vi "Velociprobe_Nanopositioner_Control_RT 2c.vi"() -> ()   [LabVIEW 2015] (continued)
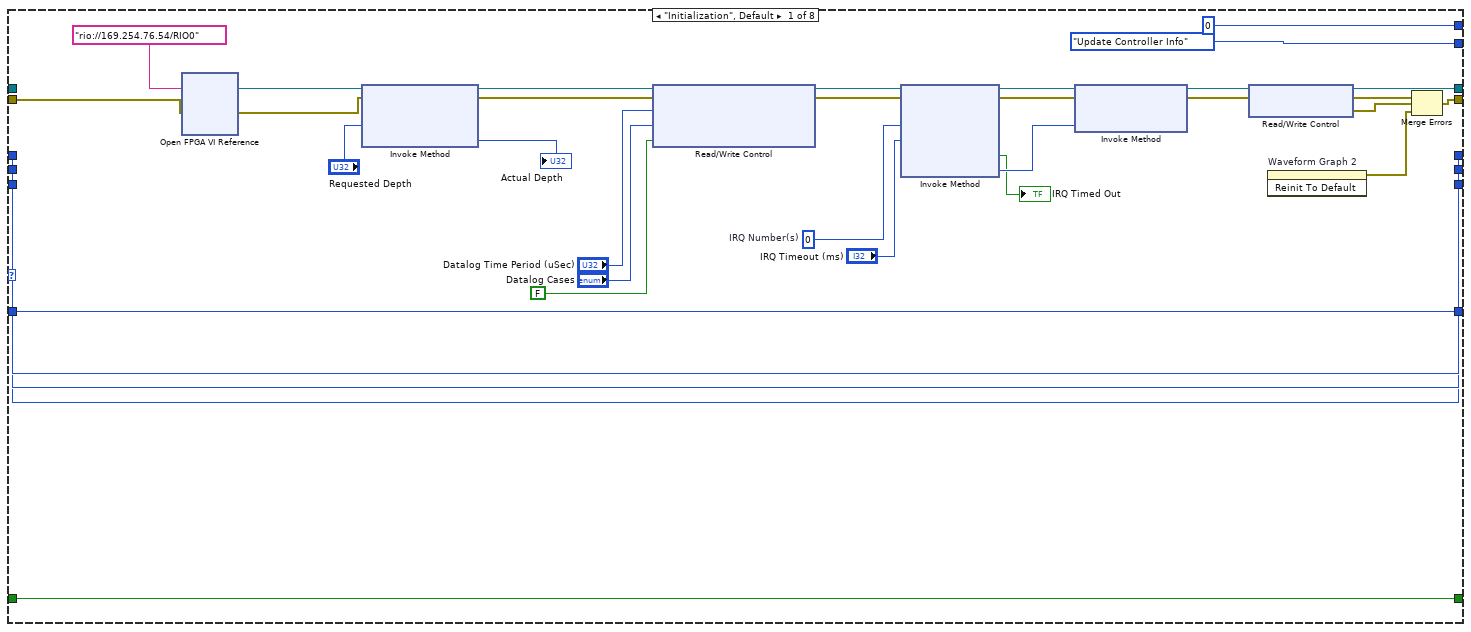
[diagram p2: hidden frame]
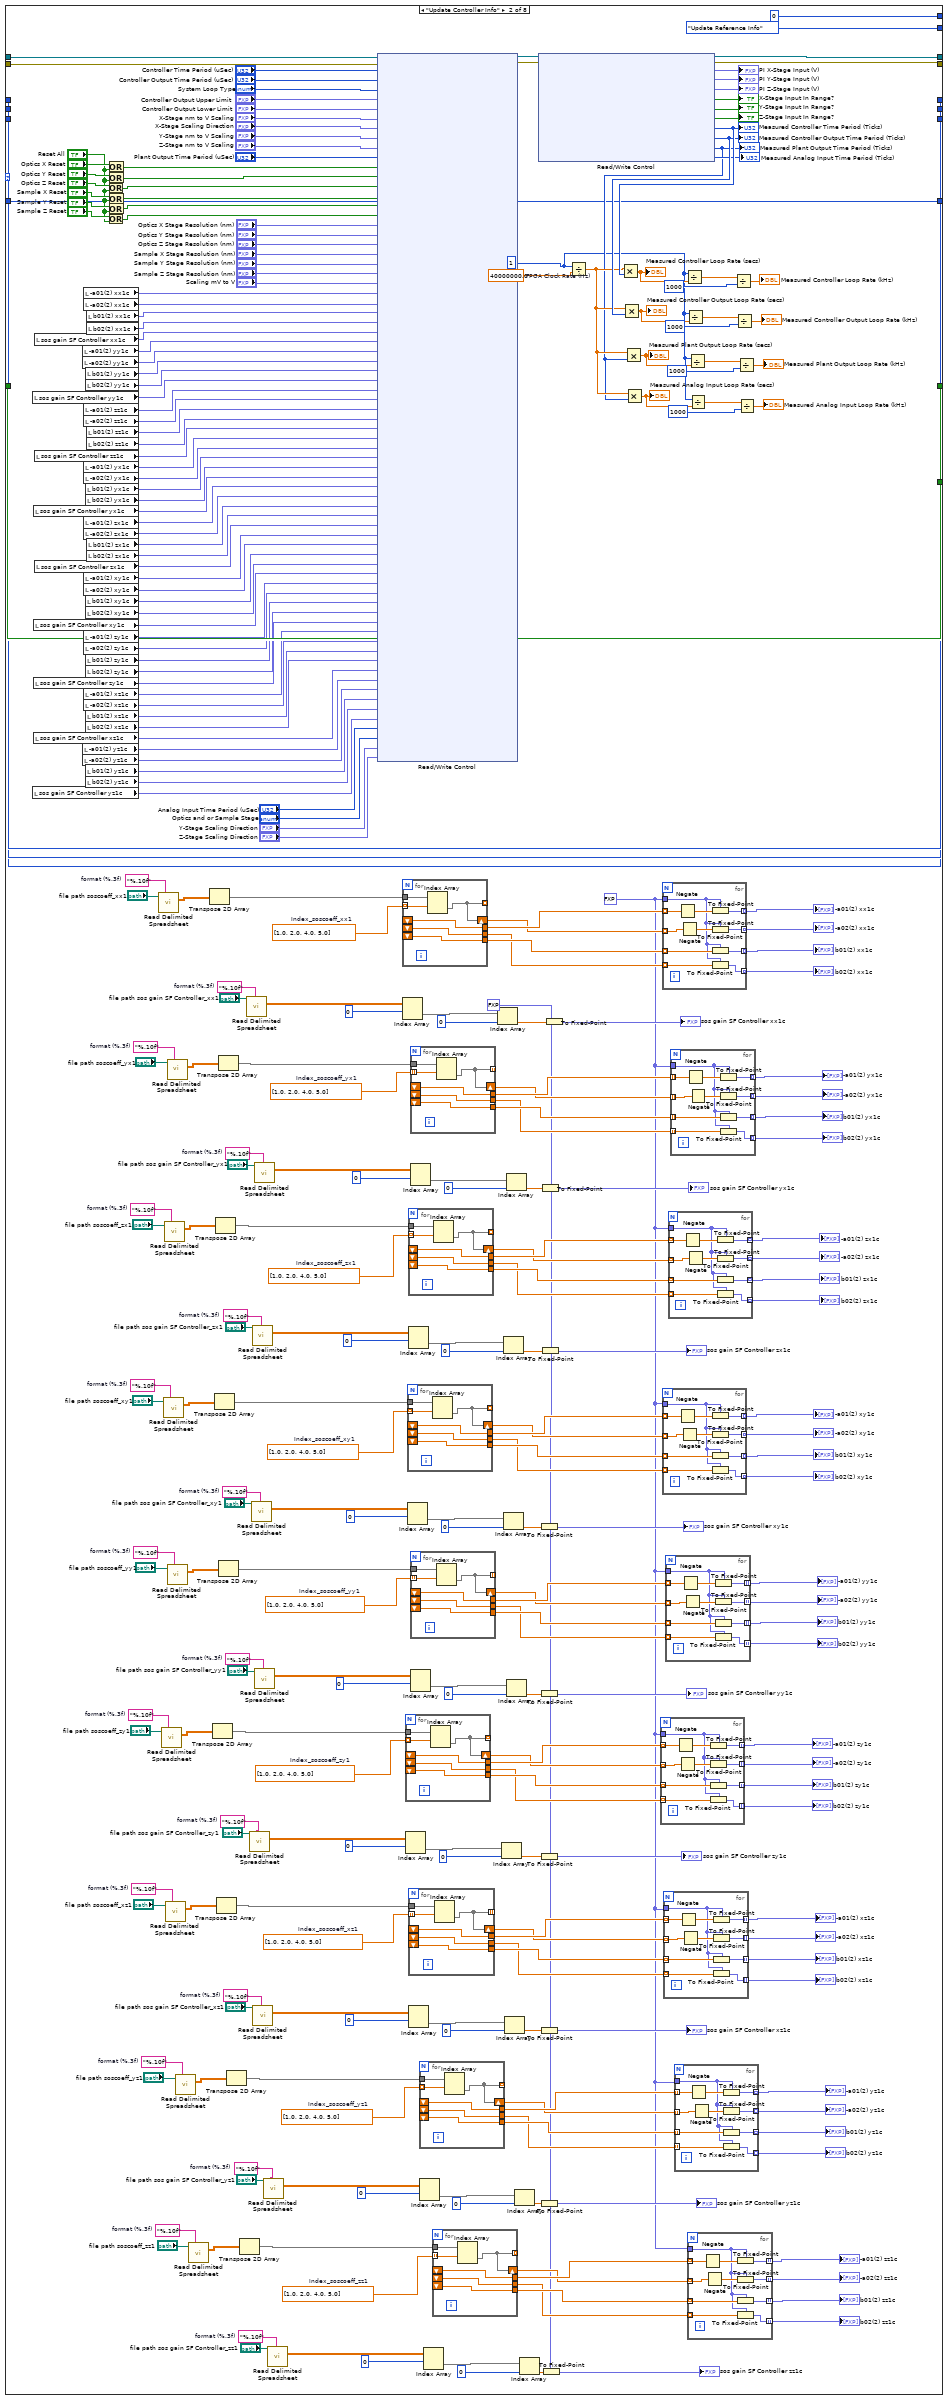
[diagram p3: hidden frame]
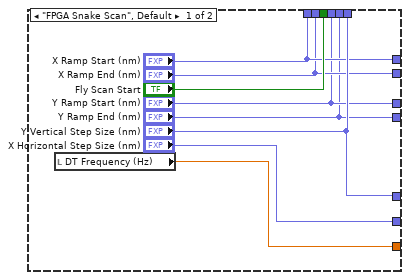
[diagram p4: hidden frame]
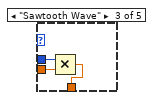
[diagram p6: hidden frame]
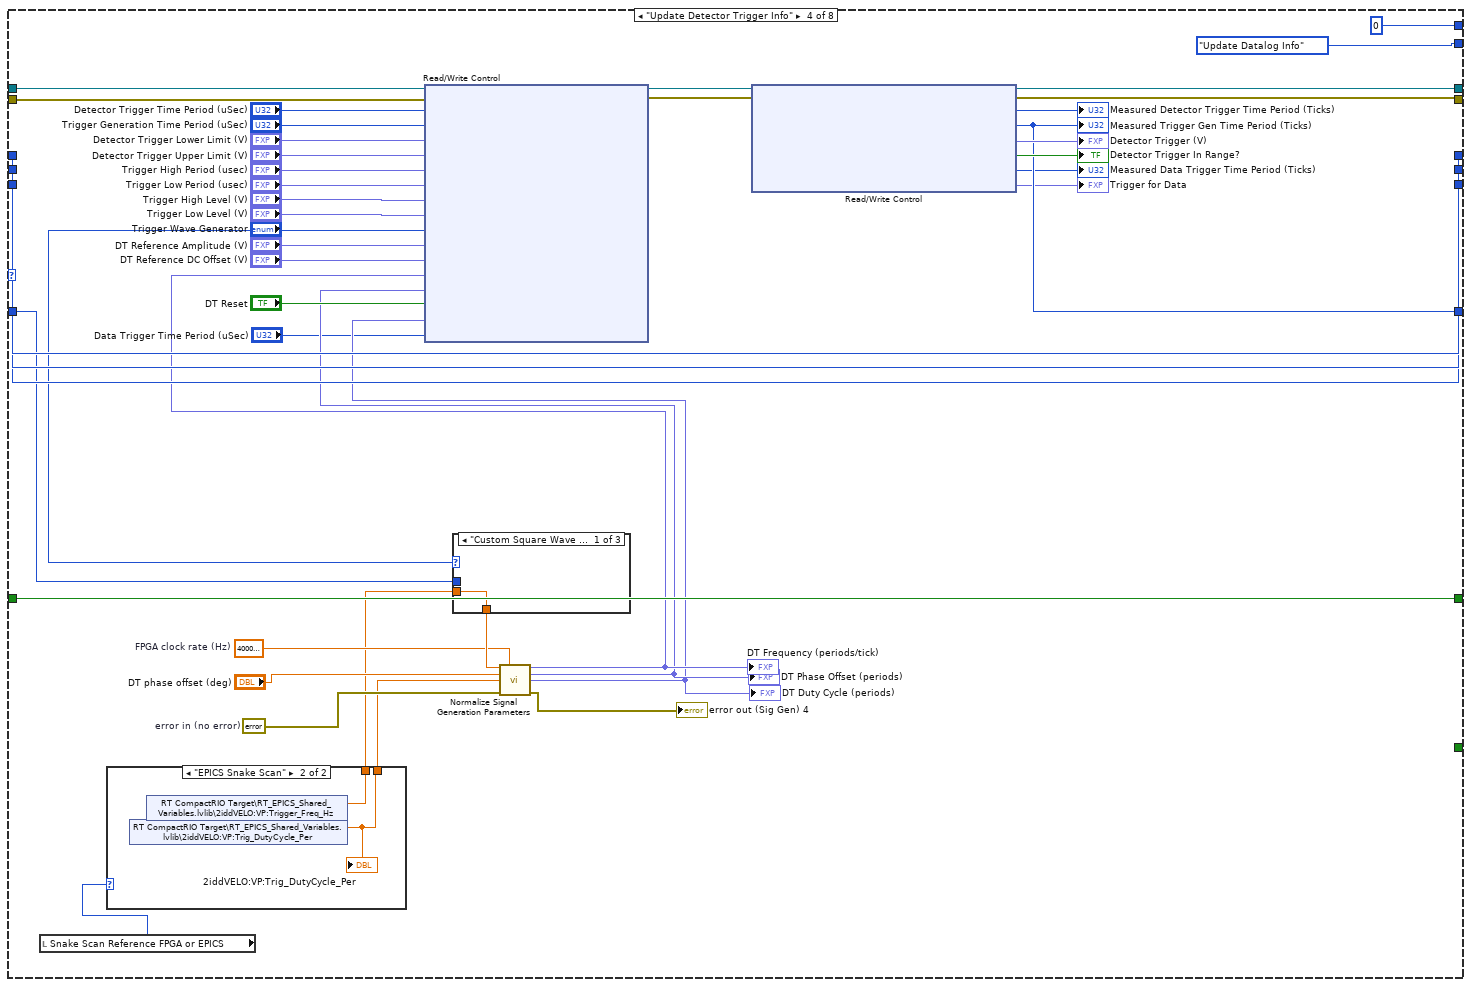
[diagram p15: hidden frame]
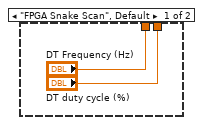
[diagram p16: hidden frame]
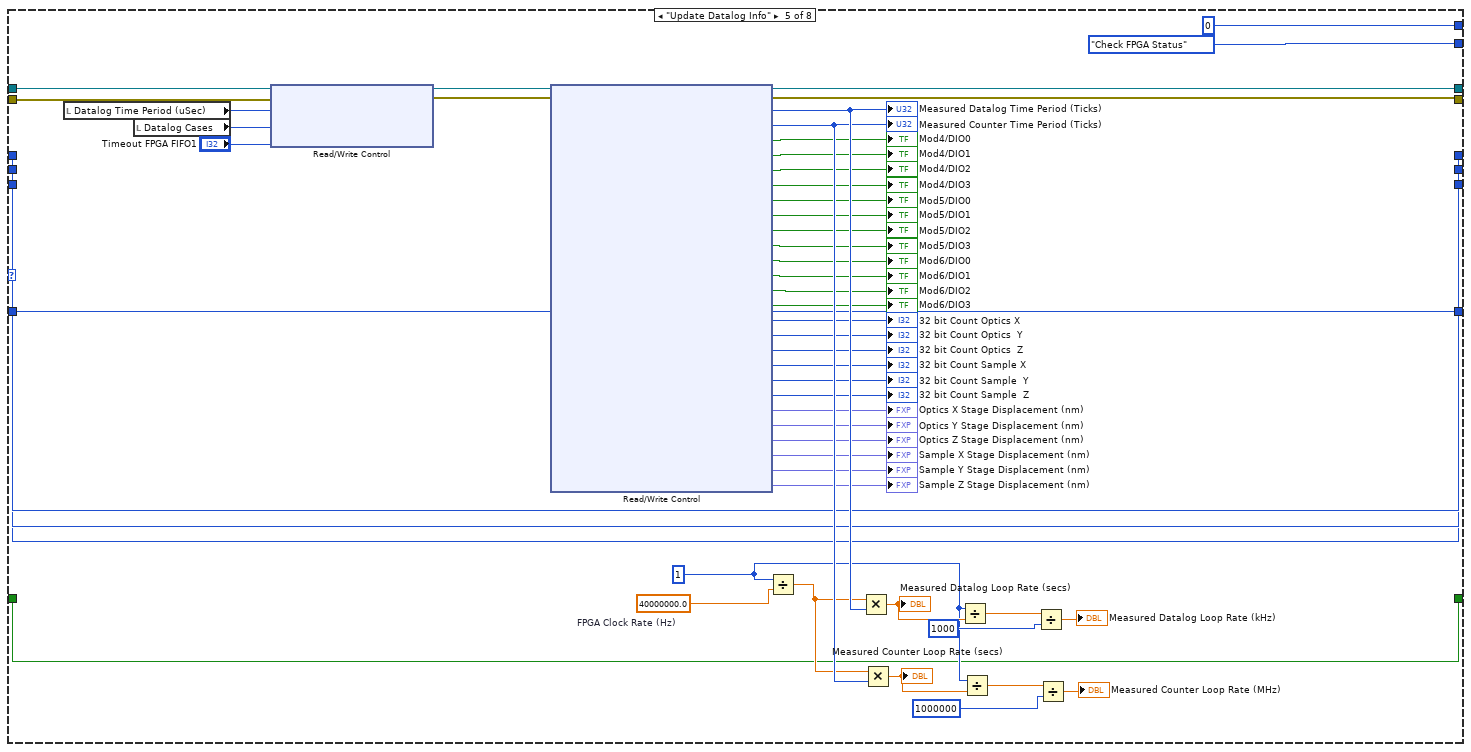
[diagram p19: hidden frame]
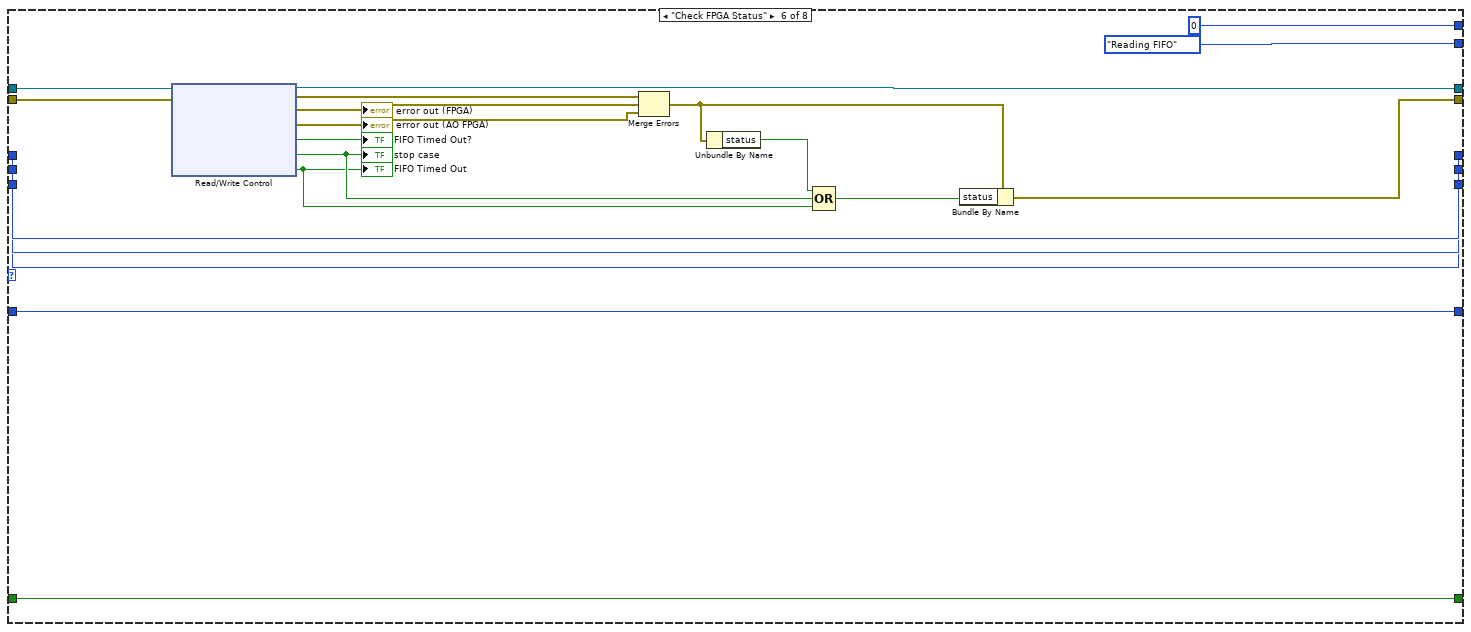
[diagram p20: hidden frame]
        }
        "-a01(2) zz1c" <- w292
        "-a02(2) zz1c" <- w291
        "b01(2) zz1c" <- w290
        "b02(2) zz1c" <- w289
        n211 = Divide(x=w81, y=w87) -> (x/y=w86:dbl)
        n212 = Divide(x=w362, y=1000) -> (x/y=→"Measured Controller Loop Rate (kHz)":dbl)
        n213 = Divide(x=w358, y=1000) -> (x/y=→"Measured Controller Output Loop Rate (kHz)":dbl)
        n214 = Divide(x=w354, y=1000) -> (x/y=→"Measured Plant Output Loop Rate (kHz)":dbl)
        n215 = Divide(x=w86, y=1000) -> (x/y=→"Measured Analog Input Loop Rate (kHz)":dbl)
      }
      frame "Update Reference Info" {
        w607 = 40000000.0  # FPGA Clock Rate (Hz)
        w601 = 1
        w614 = 40000000.0  # FPGA Clock Rate (Hz)
        w608 = 1
        w619 = errorcluster {"status"=FALSE, "code"=0, "source"=""}  # error in (no error)
        w622 = errorcluster {"status"=FALSE, "code"=0, "source"=""}  # error in (no error)
        w636 = 40000000.0  # FPGA Clock Rate (Hz)
        w630 = 1
        w648 = errorcluster {"status"=FALSE, "code"=0, "source"=""}  # error in (no error)
        w615 = 40000000.0  # FPGA clock rate (Hz)
        n216 = case shown="\"EPICS Snake Scan\"" "Snake Scan Reference FPGA or EPICS" {
          tunnel: ["X Ramp Start (nm)" w666] -> w548
          tunnel: ["X Ramp End (nm)" w665] -> w547
          tunnel: ["Fly Scan Start" w671] -> w546
          tunnel: ["Y Ramp Start (nm)" w664] -> w545
          tunnel: ["Y Ramp End (nm)" w663] -> w544
          tunnel: ["Y Vertical Step Size (nm)" w667] -> w543
          tunnel: ["X Horizontal Step Size (nm)" w670] -> w542
          tunnel: [w657 w668] -> w541
          tunnel: ["Y Vertical Step Size (nm)" w667] -> w534
          tunnel: ["X Ramp Start (nm)" w666] -> w533
          tunnel: ["X Ramp End (nm)" w665] -> w532
          tunnel: ["Y Ramp Start (nm)" w664] -> w531
          tunnel: ["Y Ramp End (nm)" w663] -> w530
          frame "FPGA Snake Scan", Default {
            n217 = local read "DT Frequency (Hz)"() -> (w657:dbl)
          }
          frame "EPICS Snake Scan" {
            w669 = fxp<+/-,16,16> 0.0 ("fixed-point type")
            n218 = shared-variable "RT CompactRIO Target\\RT_EPICS_Shared_Variables.lvlib\\2iddVELO:VP:Trigger_Freq_Hz"() -> (w668:dbl)  [unwired: 1 in, 1 out]
            "2iddVELO:VP:Trigger_Freq_Hz" <- w668
            n219 = shared-variable "RT CompactRIO Target\\RT_EPICS_Shared_Variables.lvlib\\2iddVELO:VP:Y_Step_Size_nm"() -> (w673:dbl)  [unwired: 1 in, 1 out]
            "2iddVELO:VP:Y_Step_Size_nm" <- w673
            n220 = shared-variable "RT CompactRIO Target\\RT_EPICS_Shared_Variables.lvlib\\2iddVELO:VP:X_Step_Size_nm"() -> (w672:dbl)  [unwired: 1 in, 1 out]
            "2iddVELO:VP:X_Step_Size_nm" <- w672
            n221 = shared-variable "RT CompactRIO Target\\RT_EPICS_Shared_Variables.lvlib\\2iddVELO:VP:Y_Start_nm"() -> (w674:dbl)  [unwired: 1 in, 1 out]
            n222 = shared-variable "RT CompactRIO Target\\RT_EPICS_Shared_Variables.lvlib\\2iddVELO:VP:Y_End_nm"() -> (w662:dbl)  [unwired: 1 in, 1 out]
            n223 = shared-variable "RT CompactRIO Target\\RT_EPICS_Shared_Variables.lvlib\\2iddVELO:VP:Flyscan_Start"() -> (w671:bool)  [unwired: 1 in, 1 out]
            "2iddVELO:VP:Flyscan_Start" <- w671
            n224 = shared-variable "RT CompactRIO Target\\RT_EPICS_Shared_Variables.lvlib\\2iddVELO:VP:X_Start_nm"() -> (w676:dbl)  [unwired: 1 in, 1 out]
            "2iddVELO:VP:X_Start_nm" <- w676
            n225 = shared-variable "RT CompactRIO Target\\RT_EPICS_Shared_Variables.lvlib\\2iddVELO:VP:X_End_nm"() -> (w675:dbl)  [unwired: 1 in, 1 out]
            "2iddVELO:VP:X_End_nm" <- w675
            n226 = Negate(x=w662) -> (-x=w661:dbl)
            "2iddVELO:VP:Y_End_nm" <- w661
            n227 = Negate(x=w674) -> (-x=w660:dbl)
            "2iddVELO:VP:Y_Start_nm" <- w660
            n228 = To Fixed-Point(fixed-point type=w669, number=w676) -> (fixed-point=w666:fxp<+/-,16,16>)
            n229 = To Fixed-Point(fixed-point type=w669, number=w675) -> (fixed-point=w665:fxp<+/-,16,16>)
            n230 = To Fixed-Point(fixed-point type=w669, number=w660) -> (fixed-point=w664:fxp<+/-,16,16>)
            n231 = To Fixed-Point(fixed-point type=w669, number=w661) -> (fixed-point=w663:fxp<+/-,16,16>)
            n232 = To Fixed-Point(fixed-point type=w669, number=w673) -> (fixed-point=w667:fxp<+/-,16,16>)
            n233 = To Fixed-Point(fixed-point type=w669, number=w672) -> (fixed-point=w670:fxp<+/-,16,16>)
          }
        }
        n234 = local read "X Ramp Period (usec)"() -> (w550:fxp<+,24,24>)
        n235 = local read "Y Ramp Period (usec)"() -> (w551:fxp<+,24,24>)
        n236 = case shown="\"Constant\", Default" "Z Reference Wave Selection" {
          tunnel: "Z frequency (Hz)" -> [w677 w678 w680 w682 w683]
          tunnel: [w677 w678 w679 w682 w683] -> w576
          tunnel: w575 -> [_ _ w681 _ _]
          frame "Constant", Default {
          }
          frame "Sine Wave" {
          }
          frame "Sawtooth Wave" {
            n237 = Multiply(x=w681, y=w680) -> (x*y=w679:dbl)
          }
          frame "Square Wave" {
          }
          frame "Filtered White Noise" {
          }
        }
        n238 = case shown="\"Constant\", Default" "Y Reference Wave Selection" {
          tunnel: "Y frequency (Hz)" -> [w684 w685 w686 w687]
          tunnel: [w684 w685 w686 w687] -> w581
          tunnel: w578 -> [_ _ _ _]
          frame "Constant", Default {
          }
          frame "Sine Wave" {
          }
          frame "Custom Ramp Wave" {
          }
          frame "Filtered White Noise" {
          }
        }
        n239 = case shown="\"Custom Up Down Ramp\"" "X Reference Wave Selection" {
          tunnel: "X frequency (Hz)" -> [w688 w689 w690 w691]
          tunnel: [w688 w689 w690 w691] -> w585
          tunnel: w583 -> [_ _ _ _]
          frame "Constant", Default {
          }
          frame "Sine Wave" {
          }
          frame "Custom Up Down Ramp" {
          }
          frame "Filtered White Noise" {
          }
        }
        n240 = call <vilib>:"Normalize Signal Generation Parameters.vi"("frequency (Hz)"=w581, "FPGA clock rate (Hz)"=w615, "phase offset (deg)"="Y phase offset (deg)", "error in (no error)"=w622) -> ("frequency (periods/tick)"=w618:fxp<+,32,0>, "phase offset (periods)"=w617:fxp<+,32,0>, "error out"=→"error out (Sig Gen) 2":errorcluster)  [unwired: 6 in, 3 out]
        "Y frequency (periods/tick)" <- w618
        "Y phase offset (periods)" <- w617
        n241 = call <vilib>:"Normalize Signal Generation Parameters.vi"("frequency (Hz)"=w576, "FPGA clock rate (Hz)"=w615, "phase offset (deg)"="Z phase offset (deg)", "error in (no error)"=w619) -> ("frequency (periods/tick)"=w616:fxp<+,32,0>, "phase offset (periods)"=w594:fxp<+,32,0>, "error out"=→"error out (Sig Gen) 3":errorcluster)  [unwired: 6 in, 3 out]
        "Z frequency (periods/tick)" <- w616
        "Z phase offset (periods)" <- w594
        n242 = call <vilib>:"Normalize Signal Generation Parameters.vi"("frequency (Hz)"=w585, "FPGA clock rate (Hz)"=w615, "phase offset (deg)"="X phase offset (deg)", "error in (no error)"=w648) -> ("frequency (periods/tick)"=w647:fxp<+,32,0>, "phase offset (periods)"=w625:fxp<+,32,0>, "error out"=→"error out (Sig Gen)":errorcluster)  [unwired: 6 in, 3 out]
        "X frequency (periods/tick)" <- w647
        "X phase offset (periods)" <- w625
        n243 = xnode "Read/Write Control"("FPGA VI Reference In"=w540, "error in"=w539, "X Reference Time Period (uSec)"="X Reference Time Period (uSec)", "Y Reference Time Period (uSec)"="Y Reference Time Period (uSec)", "Z Reference Time Period (uSec)"="Z Reference Time Period (uSec)", "X Reference Wave Selection"="X Reference Wave Selection", "Y Reference Wave Selection"="Y Reference Wave Selection", "Z Reference Wave Selection"="Z Reference Wave Selection", "X Reference Reset"="X Reference Reset", "Y Reference Reset"="Y Reference Reset", "Z Reference Reset"="Z Reference Reset", "X Reference Amplitude (nm)"="X Reference Amplitude (nm)", "Y Reference Amplitude (nm)"="Y Reference Amplitude (nm)", "Z Reference Amplitude (nm)"="Z Reference Amplitude (nm)", "X Frequency (periods/tick)"=w647, "X Phase Offset (periods)"=w625, "Y Frequency (periods/tick)"=w618, "Y Phase Offset (periods)"=w617, "Z Frequency (periods/tick)"=w616, "Z Phase Offset (periods)"=w594, "X Reference DC Offset (nm)"="X Reference DC Offset (nm)", "Y Reference DC Offset (nm)"="Y Reference DC Offset (nm)", "Z Reference DC Offset (nm)"="Z Reference DC Offset (nm)", "X White Noise Amplitude"="X White Noise Amplitude", "X White Noise Seed"="X White Noise Seed", "Y White Noise Amplitude"="Y White Noise Amplitude", "Y White Noise Seed"="Y White Noise Seed", "Z White Noise Amplitude"="Z White Noise Amplitude", "Z White Noise Seed"="Z White Noise Seed", "Mod 3 AI0 V to nm Scaling"="Mod 3 AI0 V to nm Scaling", "Mod 3 AI1 V to nm Scaling"="Mod 3 AI1 V to nm Scaling", "Mod 3 AI2 V to nm Scaling"="Mod 3 AI2 V to nm Scaling", "X Ramp Period (usec)"=w550, "X Ramp Start (nm)"=w548, "X Ramp End (nm)"=w547, "X Start Marker (nm)"="X Start Marker (nm)", "Fly Scan Start"=w546, "Y Ramp Period (usec)"=w551, "Y Ramp Start (nm)"=w545, "Y Ramp End (nm)"=w544, "Y Ramp Drop Size (nm)"=w543, "Y Start Marker (nm)"="Y Start Marker (nm)") -> ("FPGA VI Reference Out"=w538:refnum<k20>, "error out"=w537:errorcluster)
        n244 = xnode "Read/Write Control"("FPGA VI Reference In"=w538, "error in"=w537) -> ("FPGA VI Reference Out"=w535:refnum<k20>, "error out"=w536:errorcluster, "X Stage Reference (nm)"=→"X Stage Reference (nm)":fxp<+/-,58,25>, "Y Stage Reference (nm)"=→"Y Stage Reference (nm)":fxp<+/-,58,25>, "Z Stage Reference (nm)"=→"Z Stage Reference (nm)":fxp<+/-,58,25>, "Measured X Reference Time Period (Ticks)"=w584:u32, "Measured Y Reference Time Period (Ticks)"=w580:u32, "Measured Z Reference Time Period (Ticks)"=w579:u32, "Fly Scan Running"=→"Fly Scan Running":bool, "Continue Run"=→"Continue Run":bool)
        "Measured X Reference Time Period (Ticks)" <- w584
        "Measured Y Reference Time Period (Ticks)" <- w580
        "Measured Z Reference Time Period (Ticks)" <- w579
        n245 = Subtract(x=w531, y=w530) -> (x-y=w567:fxp<+/-,17,17>)
        n246 = Subtract(x=w533, y=w532) -> (x-y=w565:fxp<+/-,17,17>)
        n247 = Absolute Value(x=w567) -> (abs(x)=w558:fxp<+,16,16>)
        n248 = Absolute Value(x=w565) -> (abs(x)=w564:fxp<+,16,16>)
        n249 = Divide(x=w564, y=w542) -> (x/y=w562:fxp<+/-,33,17>)
        "# of Points per Line" <- w562
        n250 = Divide(x=w630, y=w636) -> (x/y=w631:dbl)
        n251 = Divide(x=w608, y=w614) -> (x/y=w609:dbl)
        n252 = Divide(x=w601, y=w607) -> (x/y=w602:dbl)
        n253 = Divide(x=w562, y=w541) -> (x/y=w554:dbl)
        "sec per line" <- w554
        n254 = Multiply(x=w631, y=w584) -> (x*y=w635:dbl)
        "Measured X Reference Loop Rate (secs)" <- w635
        n255 = Multiply(x=w609, y=w580) -> (x*y=w613:dbl)
        "Measured Y Reference Loop Rate (secs)" <- w613
        n256 = Divide(x=w558, y=w534) -> (x/y=w559:fxp<+/-,33,17>)
        n257 = Multiply(x=w602, y=w579) -> (x*y=w606:dbl)
        "Measured Z Reference Loop Rate (secs)" <- w606
        n258 = Add(x=w559, y=fxp<+,16,16> 1.0) -> (x+y=w553:fxp<+/-,34,18>)
        "# of Hor Lines" <- w553
        n259 = Multiply(x=w554, y=1000000.0) -> (x*y=w557:dbl)
        "X Ramp Period DBL (usec)" <- w557
        n260 = Reciprocal(x=w554) -> (1/x=→"line per sec (Hz)":dbl)
        n261 = Divide(x=w630, y=w635) -> (x/y=w634:dbl)
        n262 = Divide(x=w608, y=w613) -> (x/y=w612:dbl)
        n263 = To Fixed-Point(fixed-point type=fxp<+,24,24> 0.0, number=w557) -> (fixed-point=→"X Ramp Period (usec)" →"Y Ramp Period (usec)":fxp<+,24,24>)
        n264 = Multiply(x=w554, y=w553) -> (x*y=→"Total Scan Time (sec)":dbl)
        n265 = Divide(x=w601, y=w606) -> (x/y=w605:dbl)
        n266 = Multiply(x=w553, y=w562) -> (x*y=→"# Total Trigger Points":fxp<+/-,64,34>)
        n267 = Divide(x=w634, y=1000) -> (x/y=→"Measured X Reference Loop Rate (kHz)":dbl)
        n268 = Divide(x=w612, y=1000) -> (x/y=→"Measured Y Reference Loop Rate (kHz)":dbl)
        n269 = Divide(x=w605, y=1000) -> (x/y=→"Measured Z Reference Loop Rate (kHz)":dbl)
      }
      frame "Update Detector Trigger Info" {
        w710 = 40000000.0  # FPGA clock rate (Hz)
        w712 = errorcluster {"status"=FALSE, "code"=0, "source"=""}  # error in (no error)
        n270 = local read "Snake Scan Reference FPGA or EPICS"() -> (w703:enum16{"FPGA Snake Scan", "EPICS Snake Scan"})
        n271 = case shown="\"EPICS Snake Scan\"" w703 {
          tunnel: ["DT Frequency (Hz)" w738] -> w702
          tunnel: ["DT duty cycle (%)" w737] -> w701
          frame "FPGA Snake Scan", Default {
          }
          frame "EPICS Snake Scan" {
            n272 = shared-variable "RT CompactRIO Target\\RT_EPICS_Shared_Variables.lvlib\\2iddVELO:VP:Trig_DutyCycle_Per"() -> (w737:dbl)  [unwired: 1 in, 1 out]
            "2iddVELO:VP:Trig_DutyCycle_Per" <- w737
            n273 = shared-variable "RT CompactRIO Target\\RT_EPICS_Shared_Variables.lvlib\\2iddVELO:VP:Trigger_Freq_Hz"() -> (w738:dbl)  [unwired: 1 in, 1 out]
          }
        }
        n274 = case shown="\"Custom Square Wave \", Default" "Trigger Wave Generator" {
          tunnel: w702 -> [w739 w740 w741]
          tunnel: [w739 w740 w741] -> w711
          tunnel: w704 -> [_ _ _]
          frame "Custom Square Wave ", Default {
          }
          frame "Square Wave 1" {
          }
          frame "Square Wave 2" {
          }
        }
        n275 = call <vilib>:"Normalize Signal Generation Parameters.vi"("frequency (Hz)"=w711, "FPGA clock rate (Hz)"=w710, "phase offset (deg)"="DT phase offset (deg)", "duty cycle (%)"=w701, "error in (no error)"=w712) -> ("frequency (periods/tick)"=w708:fxp<+,32,0>, "phase offset (periods)"=w707:fxp<+,32,0>, "duty cycle (periods)"=w706:fxp<+,32,0>, "error out"=→"error out (Sig Gen) 4":errorcluster)  [unwired: 5 in, 2 out]
        "DT Frequency (periods/tick)" <- w708
        "DT Phase Offset (periods)" <- w707
        "DT Duty Cycle (periods)" <- w706
        n276 = xnode "Read/Write Control"("FPGA VI Reference In"=w700, "error in"=w699, "Detector Trigger Time Period (uSec)"="Detector Trigger Time Period (uSec)", "Trigger Generation Time Period (uSec)"="Trigger Generation Time Period (uSec)", "Detector Trigger Lower Limit (V)"="Detector Trigger Lower Limit (V)", "Detector Trigger Upper Limit (V)"="Detector Trigger Upper Limit (V)", "Trigger High Period (usec)"="Trigger High Period (usec)", "Trigger Low Period (usec)"="Trigger Low Period (usec)", "Trigger High Level (V)"="Trigger High Level (V)", "Trigger Low Level (V)"="Trigger Low Level (V)", "Trigger Wave Generator"="Trigger Wave Generator", "DT Reference Amplitude (V)"="DT Reference Amplitude (V)", "DT Reference DC Offset (V)"="DT Reference DC Offset (V)", "DT Frequency (periods/tick)"=w708, "DT Phase Offset (periods)"=w707, "DT Reset"="DT Reset", "DT Duty Cycle (periods)"=w706, "Data Trigger Time Period (uSec)"="Data Trigger Time Period (uSec)") -> ("FPGA VI Reference Out"=w698:refnum<k20>, "error out"=w697:errorcluster)
        n277 = xnode "Read/Write Control"("FPGA VI Reference In"=w698, "error in"=w697) -> ("FPGA VI Reference Out"=w696:refnum<k20>, "error out"=w695:errorcluster, "Measured Detector Trigger Time Period (Ticks)"=→"Measured Detector Trigger Time Period (Ticks)":u32, "Measured Trigger Gen Time Period (Ticks)"=w705:u32, "Detector Trigger (V)"=→"Detector Trigger (V)":fxp<+/-,20,5>, "Detector Trigger In Range?"=→"Detector Trigger In Range?":bool, "Measured Data Trigger Time Period (Ticks)"=→"Measured Data Trigger Time Period (Ticks)":u32, "Trigger for Data"=→"Trigger for Data":fxp<+/-,58,25>)
        "Measured Trigger Gen Time Period (Ticks)" <- w705
      }
      frame "Update Datalog Info" {
        w786 = 40000000.0  # FPGA Clock Rate (Hz)
        w775 = 1
        n278 = local read "Datalog Time Period (uSec)"() -> (w773:u32)
        n279 = local read "Datalog Cases"() -> (w772:T6)
        n280 = xnode "Read/Write Control"("FPGA VI Reference In"=w747, "error in"=w746, "Datalog Time Period (uSec)"=w773, "Datalog Cases"=w772, "Timeout FPGA FIFO1"="Timeout FPGA FIFO1") -> ("FPGA VI Reference Out"=w745:refnum<k20>, "error out"=w744:errorcluster)
        n281 = xnode "Read/Write Control"("FPGA VI Reference In"=w745, "error in"=w744) -> ("FPGA VI Reference Out"=w742:refnum<k20>, "error out"=w743:errorcluster, "Measured Datalog Time Period (Ticks)"=w785:u32, "Measured Counter Time Period (Ticks)"=w783:u32, "Mod4/DIO0"=→"Mod4/DIO0":bool, "Mod4/DIO1"=→"Mod4/DIO1":bool, "Mod4/DIO2"=→"Mod4/DIO2":bool, "Mod4/DIO3"=→"Mod4/DIO3":bool, "Mod5/DIO0"=→"Mod5/DIO0":bool, "Mod5/DIO1"=→"Mod5/DIO1":bool, "Mod5/DIO2"=→"Mod5/DIO2":bool, "Mod5/DIO3"=→"Mod5/DIO3":bool, "Mod6/DIO0"=→"Mod6/DIO0":bool, "Mod6/DIO1"=→"Mod6/DIO1":bool, "Mod6/DIO2"=→"Mod6/DIO2":bool, "Mod6/DIO3"=→"Mod6/DIO3":bool, "32 bit Count Optics X"=→"32 bit Count Optics X":i32, "32 bit Count Optics  Y"=→"32 bit Count Optics  Y":i32, "32 bit Count Optics  Z"=→"32 bit Count Optics  Z":i32, "32 bit Count Sample X"=→"32 bit Count Sample X":i32, "32 bit Count Sample  Y"=→"32 bit Count Sample  Y":i32, "32 bit Count Sample  Z"=→"32 bit Count Sample  Z":i32, "Optics X Stage Displacement (nm)"=→"Optics X Stage Displacement (nm)":fxp<+/-,58,25>, "Optics Y Stage Displacement (nm)"=→"Optics Y Stage Displacement (nm)":fxp<+/-,58,25>, "Optics Z Stage Displacement (nm)"=→"Optics Z Stage Displacement (nm)":fxp<+/-,58,25>, "Sample X Stage Displacement (nm)"=→"Sample X Stage Displacement (nm)":fxp<+/-,58,25>, "Sample Y Stage Displacement (nm)"=→"Sample Y Stage Displacement (nm)":fxp<+/-,58,25>, "Sample Z Stage Displacement (nm)"=→"Sample Z Stage Displacement (nm)":fxp<+/-,58,25>)
        "Measured Datalog Time Period (Ticks)" <- w785
        "Measured Counter Time Period (Ticks)" <- w783
        n282 = Divide(x=w775, y=w786) -> (x/y=w782:dbl)
        n283 = Multiply(x=w782, y=w785) -> (x*y=w793:dbl)
        "Measured Datalog Loop Rate (secs)" <- w793
        n284 = Multiply(x=w782, y=w783) -> (x*y=w789:dbl)
        "Measured Counter Loop Rate (secs)" <- w789
        n285 = Divide(x=w775, y=w793) -> (x/y=w792:dbl)
        n286 = Divide(x=w775, y=w789) -> (x/y=w788:dbl)
        n287 = Divide(x=w792, y=1000) -> (x/y=→"Measured Datalog Loop Rate (kHz)":dbl)
        n288 = Divide(x=w788, y=1000000) -> (x/y=→"Measured Counter Loop Rate (MHz)":dbl)
      }
      frame "Check FPGA Status" {
        n289 = xnode "Read/Write Control"("FPGA VI Reference In"=w799, "error in"=w798) -> ("FPGA VI Reference Out"=w797:refnum<k20>, "error out"=w796:errorcluster, "error out (FPGA)"=w812:errorcluster, "error out (AO FPGA)"=w811:errorcluster, "FIFO Timed Out?"=→"FIFO Timed Out?":bool, "stop case"=w806:bool, "FIFO Timed Out"=w805:bool)
        "error out (FPGA)" <- w812
        "error out (AO FPGA)" <- w811
        "stop case" <- w806
        "FIFO Timed Out" <- w805
        n290 = Merge Errors "Merge Errors"(w796, w812, w811) -> (w807:errorcluster)
        n291 = Unbundle By Name "Unbundle By Name"(w807) -> ("status"=w810:bool)
        n292 = Compound Arithmetic op=OR(w810, w806, w805) -> (w808:bool)
        n293 = Bundle By Name "Bundle By Name"(cluster=w807, "status"=w808) -> (w795:errorcluster)
      }
      frame "Reading FIFO" {
        w866 = 0.0  # t0
        n294 = local read "Snake Scan Reference FPGA or EPICS"() -> (w815:enum16{"FPGA Snake Scan", "EPICS Snake Scan"})
        n295 = xnode "Read/Write Control"("FPGA VI Reference In"=w823, "error in"=w822) -> ("FPGA VI Reference Out"=w821:refnum<k20>, "error out"=w820:errorcluster, "Number of Data Strings"=→"Number of Data Strings":i32)
        n296 = case shown="\"EPICS Snake Scan\"" w815 {
          tunnel: ["Write Data" w871] -> w852
          frame "FPGA Snake Scan", Default {
          }
          frame "EPICS Snake Scan" {
            n297 = shared-variable "RT CompactRIO Target\\RT_EPICS_Shared_Variables.lvlib\\2iddVELO:VP:Write_Data"() -> (w871:bool)  [unwired: 1 in, 1 out]
            "2iddVELO:VP:Write_Data" <- w871
          }
        }
        n298 = Greater?(x=w852, y=w851) -> (0:w848:bool)
        n299 = case shown="True" w848 {
          tunnel: w822 -> [w884 w887]
          tunnel: [w884 w888] -> w846
          frame False {
          }
          frame True {
            n300 = call "Data_Write.vi"("Command List"=Data_Write_Control."Initialize", "name"="name", "error initialize"=w887) -> ("error out"=w888:errorcluster)  [unwired: 6 in]
          }
        }
        n301 = local read "Datalog Time Period (uSec)"() -> (w864:u32)
        n302 = Less?(x=w852, y=w851) -> (x < y?=w847:bool)
        n303 = Multiply(x=1e-06, y=w864) -> (x*y=w856:dbl)
        "Datalog Time Period (sec)" <- w856
        n304 = Divide(x=1.0, y=w856) -> (x/y=w860:dbl)
        "Datalog Rate (Hz)" <- w860
        n305 = Multiply(x="FIFO Time Period", y=w860) -> (x*y=w858:dbl)
        n306 = Multiply(x=5 ("Number of Data Strings 2"), y=w858) -> (x*y=w857:dbl)
        n307 = To Unsigned Long Integer(number=w857) -> (unsigned 32bit integer=w853:u32)
        "Number of Elements" <- w853
        n308 = xnode "Invoke Method"("FPGA VI Reference In"=w821, "error in"=w820, "Number of Elements"=w853, "Timeout (ms)"="Timeout (ms)") -> ("FPGA VI Reference Out"=w819:refnum<k20>, "error out"=w818:errorcluster, "Data"=w854:fxp<+/-,58,25>[], "Elements Remaining"=→"Elements Remaining" →"Elements Remaining Waveform Chart" →"Elements Remaining Waveform Chart 3":u32)
        "Data" <- w854
        n309 = Decimate 1D Array "Decimate 1D Array"(w854) -> (w837:fxp<+/-,58,25>[], w828:fxp<+/-,58,25>[], w827:fxp<+/-,58,25>[], w826:fxp<+/-,58,25>[], w824:fxp<+/-,58,25>[])
        n310 = Build Array "Build Array"(w837, w828, w827, w826, w824) -> (w867:fxp<+/-,58,25>[][])
        n311 = To Double Precision Float(number=w867) -> (double precision float=w862:dbl[][])
        n312 = call "Convert to Dynamic Data"("Array"=w837) -> ("Dynamic Data Type"=w835:dynamicdata)  [unwired: 3 in]
        n313 = call "Convert to Dynamic Data2"("Array"=w828) -> ("Dynamic Data Type"=w829:dynamicdata)  [unwired: 3 in]
        n314 = call "Convert to Dynamic Data3"("Array"=w827) -> ("Dynamic Data Type"=w831:dynamicdata)  [unwired: 3 in]
        n315 = call "Convert to Dynamic Data4"("Array"=w826) -> ("Dynamic Data Type"=w830:dynamicdata)  [unwired: 3 in]
        n316 = Transpose 2D Array(2D array=w862) -> (transposed array=w844:dbl[][])
        n317 = case shown="True" w852 {
          tunnel: w846 -> [w876 w882]
          tunnel: [w876 w883] -> w845
          tunnel: w844 -> [_ w877]
          frame False {
          }
          frame True {
            w880 = "%8f"  # format string
            w879 = ","  # delimiter (Tab)
            n318 = Array To Spreadsheet String(delimiter (Tab)=w879, array=w877, 3:w880) -> (spreadsheet string=w878:string)
            n319 = call "Data_Write.vi"("Command List"=Data_Write_Control."Write", "Data"=w878, "error initialize"=w882) -> ("error out"=w883:errorcluster)  [unwired: 6 in]
          }
        }
        n320 = call "Convert from Dynamic Data"("Dynamic Data Type"=w835) -> ("Array"=w836:dbl[])  [unwired: 3 in]
        n321 = call "Convert from Dynamic Data2"("Dynamic Data Type"=w829) -> ("Array"=w834:dbl[])  [unwired: 3 in]
        n322 = call "Convert from Dynamic Data3"("Dynamic Data Type"=w831) -> ("Array"=w833:dbl[])  [unwired: 3 in]
        n323 = call "Convert from Dynamic Data4"("Dynamic Data Type"=w830) -> ("Array"=w832:dbl[])  [unwired: 3 in]
        n324 = Bundle("Array"=w836, "Array"=w834) -> (→"XY Graph":cluster{"Array":dbl[], "Array":dbl[]})  [unwired: 1 in]
        n325 = Bundle("Array"=w833, "Array"=w832) -> (→"XY Graph 2":cluster{"Array":dbl[], "Array":dbl[]})  [unwired: 1 in]
        n326 = case shown="True" w847 {
          tunnel: w845 -> [w872 w874]
          tunnel: [w872 w875] -> w855
          frame False {
          }
          frame True {
            n327 = call "Data_Write.vi"("Command List"=Data_Write_Control."Close", "error initialize"=w874) -> ("error out"=w875:errorcluster)  [unwired: 7 in]
          }
        }
        n328 = Bundle("t0"=w866, w856, w862) -> (→"Waveform Graph 2":cluster{"t0":dbl, dbl, dbl[][]})  [unwired: 1 in]
        n329 = Merge Errors "Merge Errors"(w818, w855) -> (w817:errorcluster)
      }
      frame "Exit" {
        w901 = TRUE ("Stop")
        n330 = xnode "Invoke Method"("FPGA VI Reference In"=w895, "error in"=w894) -> ("FPGA VI Reference Out"=w893:refnum<k20>, "error out"=w892:errorcluster)
        n331 = xnode "Read/Write Control"("FPGA VI Reference In"=w893, "error in"=w892, "stop case"=TRUE) -> ("FPGA VI Reference Out"=w891:refnum<k20>, "error out"=w890:errorcluster)
        n332 = local write "Stop"(w901) -> ()
        n333 = xnode "Close FPGA VI Reference"("FPGA VI Reference In"=w891, "error in"=w890) -> ("error out"=w889:errorcluster)
      }
    }
    n334 = call "State Control.vi"("Error Input"=w14, "Input States"=w25, "Stop"="Stop") -> ("Output State"=w24:T7)  [unwired: 8 in]
    n335 = node-c288(w31) -> ()  [unwired: 1 out]
  }
  n336 = node-c288(w7) -> (→"Error (RT)":errorcluster, →"Iteration Duration RT Timed-Loop":i64)
  n337 = call <vilib>:"Simple Error Handler.vi"("error in (no error)"=w1) -> ("message"=→"message":string)  [unwired: 4 in, 4 out]
